vi "01 Dryer_Performance_SM.vi"() -> ()   [LabVIEW 2012]
uses:
  <vilib>/Platform/fileVersionInfo.llb/FileVersionInformation.ctl
  Equipment DPT.ctl
  WT500/Dryer PowerData.ctl
  Q Dryer Data.ctl
  DPT Global Type.ctl
  RMC Calc Inputs.ctl
  WT500/WT500 Sequences.ctl
  Chroma/Chroma Driver Select.ctl
  Dryer Wilt/Dryer Commands.ctl
  Nufi/Nufi Global_ReceivedDataCluster.vi
  Global Test Variables DPT.vi
  <vilib>/Analysis/baseanly.llb/Mean (DBL).vi
  <vilib>/Utility/file.llb/Write To Spreadsheet File (string).vi
  Drivers/Agilent 34970/Agilent 34970.lvlib
  <vilib>/Analysis/NI_AALBase.lvlib
panel:
  out "Low Power Switch":bool=TRUE
  out "Error Message 3":string
  out "Error Message 2":string
  in  "stop!":bool
  out "Tsamp(s)":dbl
  out "Temp OOR":bool
  in  "stop":bool
  in  "End Test Button":bool
  out "Data Filename":string
  in  "Tab Control":T1(tab)=enum."                           RMC  "
  in  "None":bool
  in  "All":bool
  out "Plot All":cluster{dbl[], dbl[]}[](graph)
  in  "Plot Legend":T2(array[cluster])
  out "2015?":bool
  out "Ave Gas Pressure":dbl format="%0.2f"
  out "Plot Power":cluster{dbl[], dbl[]}[](graph)
  out "PowerData":T3={"Current L1"=236.2, "Current L2"=17.749, "Power"=4192.0, "WattHours"=0.0}
  out "Power On":bool
  out "WH_0":dbl
  out "Wbouy":dbl
  out "Plot RMC":cluster{dbl[], dbl[]}[](graph)
  out "BDW - Bone Dry Wt(lbs)":dbl
  out "Empty Dryer Cold Weight":dbl
  out "Wet Clothing Weight":dbl
  out "Scale (LBS)":dbl
  out "RMC%":dbl=100.0
  out "Room Ambient F":dbl
  out "RDB F":dbl
  out "Cloth Weight(est.)":dbl
  out "Experimental Completion Time Estimate":dbl format="%<%H:%M:%S>t"
  out "Use Smoothing":bool=TRUE
  in  "Apply Load Offset":bool
  in  "Tab Control 2":enum32{"Debug Only", "Running"}(tab)
  in  "Debug Info":T4(tab)=enum."Settings"
  out "FileName DataLog":path caption="FileName"
  out "FileVersionInfo Out":T5
  out "Ver.":string="Development"
  out "Work File Directory":path=path "c:/Work"
  out "Number of TCs":i32
  in  "Close when complete":bool
  in  "DC Voltages Filename":path=path "c:/data/voltages.csv"
  out "Stream DC to File?":bool
  out "zip path":path
  out "Nufi Data File Path":path
  in  "Nufi?":bool=TRUE
  out "Filename Prefix String":string
  out "DOE Filename":path
  out "Error Log":errorcluster[](array[cluster])
  out "# elements in queue":i32
  out "Error Count":dbl
  out "error out":errorcluster
  out "Power Off Check":bool[](array[boolean])
  in  "Error Log 2":errorcluster[](array[cluster])
  out "Power Off Time(samples)":i32=15
  out "3011 resistor":dbl=267.4
  in  "UI Timer":i32=1000
  in  "DAQ Timer":i32=1000
  in  "Clear Graph":bool
  out "Use SL9200 Gas Readings?":bool
  in  "Simulate":bool
  in  "Supply Voltage:":string(combo)
  out "Equipment":T6
  out "Time Limit(s)":dbl=5400.0 format="%<%H:%M:%S>t"
  out "RMC Limit":dbl=2.0
  out "Enable Time Limit":bool
  out "Enable RMC Limit":bool
  in  "Weight Offset":dbl
  in  "MA Filter Size":i32=10
  in  "USB Weight?":bool=TRUE
  in  "Power On Threshold":dbl=50.0
  in  "Scale Temp Coeff":dbl
  out "Init Scale Temp":dbl=72.0
  out "3010 resistor":dbl=267.4
  out "Use Dry Gas Meter?":bool=TRUE
  out "Load Offset":dbl
  in  "Drum Volume":dbl=6.0
  out "Enable Stop On Power Off":bool=TRUE
  out "exe?":bool
  out "RMC Calc Inputs":T7
  out "Tend?":dbl format="%<%H:%M:%S>t"
  in  "W.Samps":i32=10
  out "1020 resistor":dbl=267.4
  in  "Auto Scale Reading":bool=TRUE
  out "Scale Com Port":refnum<visa-resource-name>="COM1"
  out "ITHX RH Sensor":bool
  out "Offset":dbl
  out "Init Offset Coeff":dbl
  in  "Power off Check RMC sec":dbl=7.0
  out "End4_Nufi":bool=TRUE
  out "Debug Mode":bool=TRUE
  out "Debug List Test States":string[](array[string])
  out "daq debug array":string[](array[string])
  out "UI States":string[](array[string])
  out "End1_Main":bool=TRUE
  out "Write to File":bool=TRUE
  out "Test Complete?":bool
  out "Loggin Data":bool
  out "End2_DAQ":bool=TRUE
  out "Eng3_Log":bool=TRUE
  out "BTUF3":string[][](array[string])
  out "Power On One Shot":bool
  out "Start Time (sec)":dbl format="%<%H:%M:%S>t"
  out "End Msg":string
  out "Final User Message":string="Premature Completion."
  out "cDAQ":bool=TRUE
  in  "cDAQ Setting":bool=TRUE
  out "End_End":bool=TRUE
  out "CDAQ Tasks":refnum<k21>[](array[refnum])
  out "[Temp (F), RH]":dbl[](array[numeric])
  out "Power Off One Shot":bool
  out "TC Chanel List":string
  out "DAQ Chanel List":string
  out "DAQ Label List":string[](array[string])
  out "Agilent Error Message":string
  out "DAQ Delay Time":i32
  in  "Get Data Interrupt":bool
  out "DAQ Data":dbl[](array[numeric])
  out "In Range?":bool[](array[boolean])
  in  "NPLC Value(6:1PLC)":T8(ring)=enum."1 PLC"
  in  "Channel Delay (sec)":dbl=0.01 format="%#_6e"
  in  "Channel Delay Auto (T:Enabled)":bool=TRUE
  in  "Autozero (0:ON)":enum16{"On", "Off", "Once"}(ring)
  in  "TC Check Enable (F:Disable)":bool=TRUE
  out "CDAQ Data Out":dbl[](array[numeric])
  out "Use Chroma":bool
  out "Globals for Dryer Performance Test":T9={"Test Setup"={"RH Resistor"=267.4, "Temp Cal"=72.0, "Temp Coeff"=-0.0234, "Power On Threshold"=50.0, "MA Filter Size"=60, "Weight Offset"=0.0, "Temp Resistor"=267.4, "Gas Enabled"=FALSE, "Gas P. Resistor"=250.0, "Scale Com"=1.0, "W. Samps"=5, "Temp4mA Val"=267.4, "Temp20mA Val"=267.4, "RH4mA Val"=0.0, "RH20mA Val"=100.0, "GPres4mA Val"=0.0, "Gpres20mA Val"=50.0, "Smoothing"=FALSE, "CDAQ"=FALSE, "34970"=FALSE, "34980"=FALSE, "RH-IP"="192.168.1.161", "RH-IP2"="192.168.1.161", "RH-IP3"="192.168.1.161", "CompVolume"=0.0, "T45_Coeff."=0.0}, "Agilent Setup"={"Scale Channel"="3009", "TC Channels"="1001:1040,2001:2040", "VDC Discrete Channels"="3001:3008", "RH Chan"="3010,3011", "Temp Chan"="3010,3011", "Tscale Channel"="", "RDB Channel"="1001", "Gas Temperature"="1019", "Gas Pressure"="1020", "Barometric Pressure"="1040", "Gas Feedback Chan"="3012"}, "Directories"={"Work File Directory"=path "c:/Work", "Save File Directory"=path "c:/Data", "Library Directory"=path "c:/Data", "Data Backup Directory"=path "c:/Data", "Data Backup Dir Fail"=path "c:/Data", "Lab Directory"=path "c:/Data"}, "Test Information"={"Model:"="DGnn", "Temperature:"="Mode: EHEAT", "Engineer:"="CraigT.", "Technician:"="RonR.", "Comments:"="R134A Charge Level: 50g", "Lab ID:"="DGnn", "TR Number:"="T000000", "Test Number:"="T000000", "Test Station:"="Unitialized", "Empty Dryer Cold Weight:"=0.0, "Serial Number:"="DGnn", "Build:"="DGnn", "Dryer Type"="RonR.", "Humidity"="70,50", "Test Title per TR:"="70,50"}, "cDAQ Array Locations"={"Scale Channel"="90", "TC Channels"="1-15, 65,66,67\n16-31, 68,69\n32-47, 70,71\n48-64, 72, 73", "VDC Discrete Channel"="1020,1040,3001:3008", "RH Chan"="91", "Temp Chan"="93", "Tscale Channel"="3", "RDB Channel"="1", "Gas Temperature"="0", "Gas Pressure"="89", "Barometric Pressure"="94", "Gas Feedback Chan"="92"}}
  out "Data":string[][](array[string])
  out "Power Label":string[](array[string])=["VL1", "VL2", "IL1", "IL2", "P", "WH", "Ipeak", "Phi(1,2)"]
  out "Q Element":T10
  in  "Start Test":bool
  out "Elapsed Time":dbl format="%<%H:%M:%S>t"
  out "Status Message":string
  # "Weight(Lbs)\nPower (Watts)\nCurrent (Amps)\nTemp(F)\nPressure (PSIA)\nRH (%)"
  # "(A)"
  # "(A)"
  # "(Watts)"
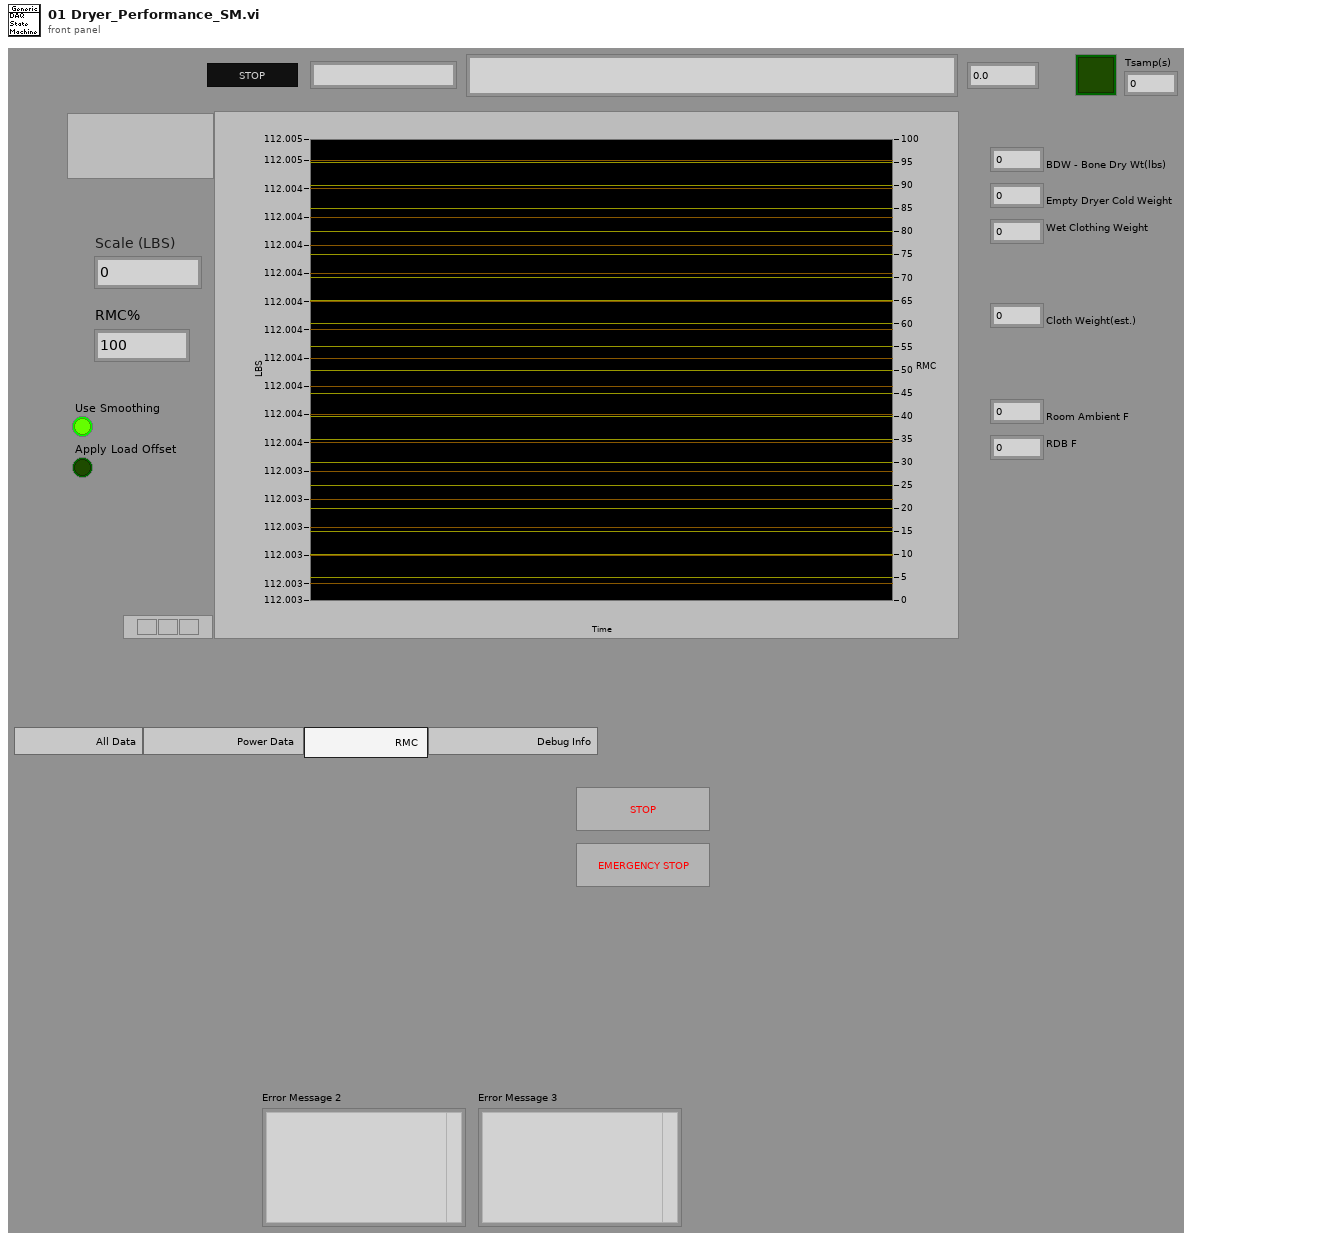
[diagram p1: front panel]
types:
  T1 = enum32{"                         All Data", "                            Power Data  ", "                           RMC  ", "                                  Debug Info"}
  T2 = cluster{"Title":string, "OnOff":bool, "Color Box":u32, "Value":dbl}[]
  T3 = typedef "Dryer PowerData.ctl" = cluster{"Current L1":dbl, "Current L2":dbl, "Power":dbl, "WattHours":dbl}
  T4 = enum32{"File Info", "Error Data", "Settings", "Test States", "Agilent Data", "Globals"}
  T5 = typedef "FileVersionInformation.ctl" = cluster{"FileVersion":string, "ProductName":string, "InternalName":string, "CompanyName":string, "LegalCopyright":string, "FileDescription":string}
  T6 = typedef "Equipment DPT.ctl" = cluster{"Com Agilent":refnum<visa-resource-name>, "Com Flow Computer":refnum<visa-resource-name>, "Com Power Meter":refnum<visa-resource-name>, "Com Power Supply":refnum<visa-resource-name>}
  T7 = typedef "RMC Calc Inputs.ctl" = cluster{"Measeured Weight":dbl, "BDW - Bone Dry Wt(lbs)":dbl, "Empty Dryer Cold Weight":dbl, "Measured IMC":dbl, "Tamb":dbl, "T-RDB":dbl, "Drum Volume":dbl, "Load Offset":dbl, "Temp Coeff":dbl, "Temp Cal":dbl, "Tscale":dbl}
  T8 = enum16{"0.02 PLC", "0.2 PLC", "1 PLC", "2 PLC", "10 PLC", "20 PLC", "100 PLC", "200 PLC"}
  T9 = typedef "DPT Global Type.ctl" = cluster{"Test Setup":cluster{"RH Resistor":dbl, "Temp Cal":dbl, "Temp Coeff":dbl, "Power On Threshold":dbl, "MA Filter Size":i32, "Weight Offset":dbl, "Temp Resistor":dbl, "Gas Enabled":bool, "Gas P. Resistor":dbl, "Scale Com":dbl, "W. Samps":i32, "Temp4mA Val":dbl, "Temp20mA Val":dbl, "RH4mA Val":dbl, "RH20mA Val":dbl, "GPres4mA Val":dbl, "Gpres20mA Val":dbl, "Smoothing":bool, "CDAQ":bool, "34970":bool, "34980":bool, "RH-IP":string, "RH-IP2":string, "RH-IP3":string, "CompVolume":dbl, "T45_Coeff.":dbl}, "Agilent Setup":cluster{"Scale Channel":string, "TC Channels":string, "VDC Discrete Channels":string, "RH Chan":string, "Temp Chan":string, "Tscale Channel":string, "RDB Channel":string, "Gas Temperature":string, "Gas Pressure":string, "Barometric Pressure":string, "Gas Feedback Chan":string}, "Directories":cluster{"Work File Directory":path, "Save File Directory":path, "Library Directory":path, "Data Backup Directory":path, "Data Backup Dir Fail":path, "Lab Directory":path}, "Test Information":cluster{"Model:":string, "Temperature:":string, "Engineer:":string, "Technician:":string, "Comments:":string, "Lab ID:":string, "TR Number:":string, "Test Number:":string, "Test Station:":string, "Empty Dryer Cold Weight:":dbl, "Serial Number:":string, "Build:":string, "Dryer Type":string, "Humidity":string, "Test Title per TR:":string}, "cDAQ Array Locations":cluster{"Scale Channel":string, "TC Channels":string, "VDC Discrete Channel":string, "RH Chan":string, "Temp Chan":string, "Tscale Channel":string, "RDB Channel":string, "Gas Temperature":string, "Gas Pressure":string, "Barometric Pressure":string, "Gas Feedback Chan":string}}
  T10 = typedef "Q Dryer Data.ctl" = cluster{"Data Array":dbl[], "Label Array":string[], "Date":string}
  T11 = enum32{"invalid app kind", "Development System", "Run Time System", "Student Edition", "Embedded LabVIEW", "Evaluation", "Custom"}
  T12 = typedef "WT500 Sequences.ctl" = enum16{"Initialize", "GetReadings", "GetErrors", "Close", "NoOp", "MiscCmd"}
  T13 = enum16{"DC Volts", "2-Wire Resistance", "4-Wire Resistance", "DC Current", "Temperature"}
  T14 = enum16{"B-Type", "E-Type", "J-Type", "K-Type", "N-Type", "R-Type", "S-Type", "T-Type"}
  T15 = enum16{"2252", "5000", "10000", "Default (Last)"}
  T16 = enum16{"100 mV", "1 V", "10 V", "100 V", "300 V", "Minimum", "Maximum"}
  T17 = cluster{"Thermocouple Type (Last)":enum16{"B", "E", "J", "K", "N", "R", "S", "T", "Default (Last)"}, "TC Rjunction (2:Int)":enum16{"Fixed", "External", "Internal"}, "Fixed Rjunction Temp (0:Manual)":enum16{"Manual", "Minimum", "Maximum"}, "TC Auto Check? (F:Don't Check)":bool, "Rjunct Temp Value (0)":dbl}
  T18 = enum16{"Exe", "Init CDAQ", "Gather DATA", "Close"}
  T19 = typedef "Chroma Driver Select.ctl" = enum16{"Initialize", "Output On 120", "Output On 240", "Output On 208", "Output Off", "Status", "Send Command", "Track Current"}
  T20 = enum16{"100 mV", "1 V", "10 V", "100 V", "300 V", "Auto", "Minimum", "Maximum", "Default"}
  T21 = enum32{"Invalid", "Standard", "Closed", "Hidden", "Minimized", "Maximized"}
  T22 = cluster{"Core":cluster{"Current VI Reference":refnum<vi>, "Close Panel on Exit?":bool}, "Error Log":errorcluster[], "FileName":path, "Config File Path":path, "Equipment":T6, "DAQ Chan List":string, "DAQ Label List":string[], "Supply Voltage:":string, "Empty Dryer Cold Weight":dbl, "Start Header Data":string[][], "Dryer Type":string, "Dryer Load Nominal Weight":string}
  T23 = typedef "DOE Audit Data.ctl" = cluster{"Technician":string, "Date":string, "Model":string, "Serial":string, "Total Dry Time(m)":dbl, "Bone Dry Wt":dbl, "Initial Wt":dbl, "Final Wt":dbl, "Initial Ret":dbl, "Final Ret":dbl, "Elect Energy Used":dbl, "Gas Meter Temp":dbl, "Gas Meter Pres":dbl, "Gas Volume":dbl, "Barometer Temp":dbl, "Barometer Pres":dbl, "Gas Corr Fact":dbl, "Cor Gas Vol":dbl, "Gas Heat Val":dbl, "Gas Energy BTU":dbl, "Gas Energy kwh 4%":dbl, "Elect Energy kwh 4%":dbl, "Total  Energy 4%":dbl, "Gas Vol Init":dbl, "Gas Vol Fin":dbl, "Start Time(s)":dbl, "End Time(s)":dbl, "Elect Energy Start":dbl, "Elect Energy End":dbl, "Per Cycle Efficency":dbl, "Annual Consumption":dbl, "Load Cycles":string, "Ambinet Temp":string, "Ambinet RH":string, "Per Cycle Off Mode/Standby Power":dbl, "Total Energy (Gas + Elect)":dbl, "Combined Energy Factor":dbl, "Off Mode Power":dbl, "Exhaust":string, "Washer Water Temperature ( 60 ± 5°F )":string, "Supply Voltage":string, "Reference Temperature (F)":string, "Reference Pressure (psi)":string, "Standby Power":dbl}
  T24 = enum16{"100 mV", "1 V", "10 V", "100 V", "300 V", "Auto", "Minimum", "Maximum"}
  T25 = typedef "Dryer Commands.ctl" = u8
  T26 = cluster{"[Temp (F), RH][0]":dbl, "[Temp (F), RH][1]":dbl}
  T27 = cluster{"Measured IMC":dbl, "Actual RMC":dbl, "RMC (Desired)":dbl, "Bone Dry Wt(lbs)":dbl, "Tolerance(%)":dbl}
  T28 = cluster{"Current VI Reference":refnum<vi>, "Close Panel on Exit?":bool}
  T29 = cluster{"queue out":refnum<queue>, "Q Element":T10, "Graph Reset":bool, "Init Save File":bool, "Time Array":dbl[], "Data Array":dbl[][], "Enable RMC":bool, "Power Previous":bool}
  T30 = cluster{"Title":string, "OnOff":bool, "Color Box":u32, "Value":dbl}
  T31 = cluster{"[0]":dbl, "[1]":dbl, "[2]":dbl, "[3]":dbl, "[4]":dbl, "[5]":dbl}
  T32 = cluster{"[0]":dbl, "[1]":dbl, "[2]":dbl, "[3]":dbl}
  T33 = enum16{"Left Button", "Center Button", "Right Button", "Window Close"}
  T34 = cluster{"queue out":refnum<queue>, "Q Element":T10, "Equipment":T6, "DAQ Chanel List":string, "Error Log 2":errorcluster[]}
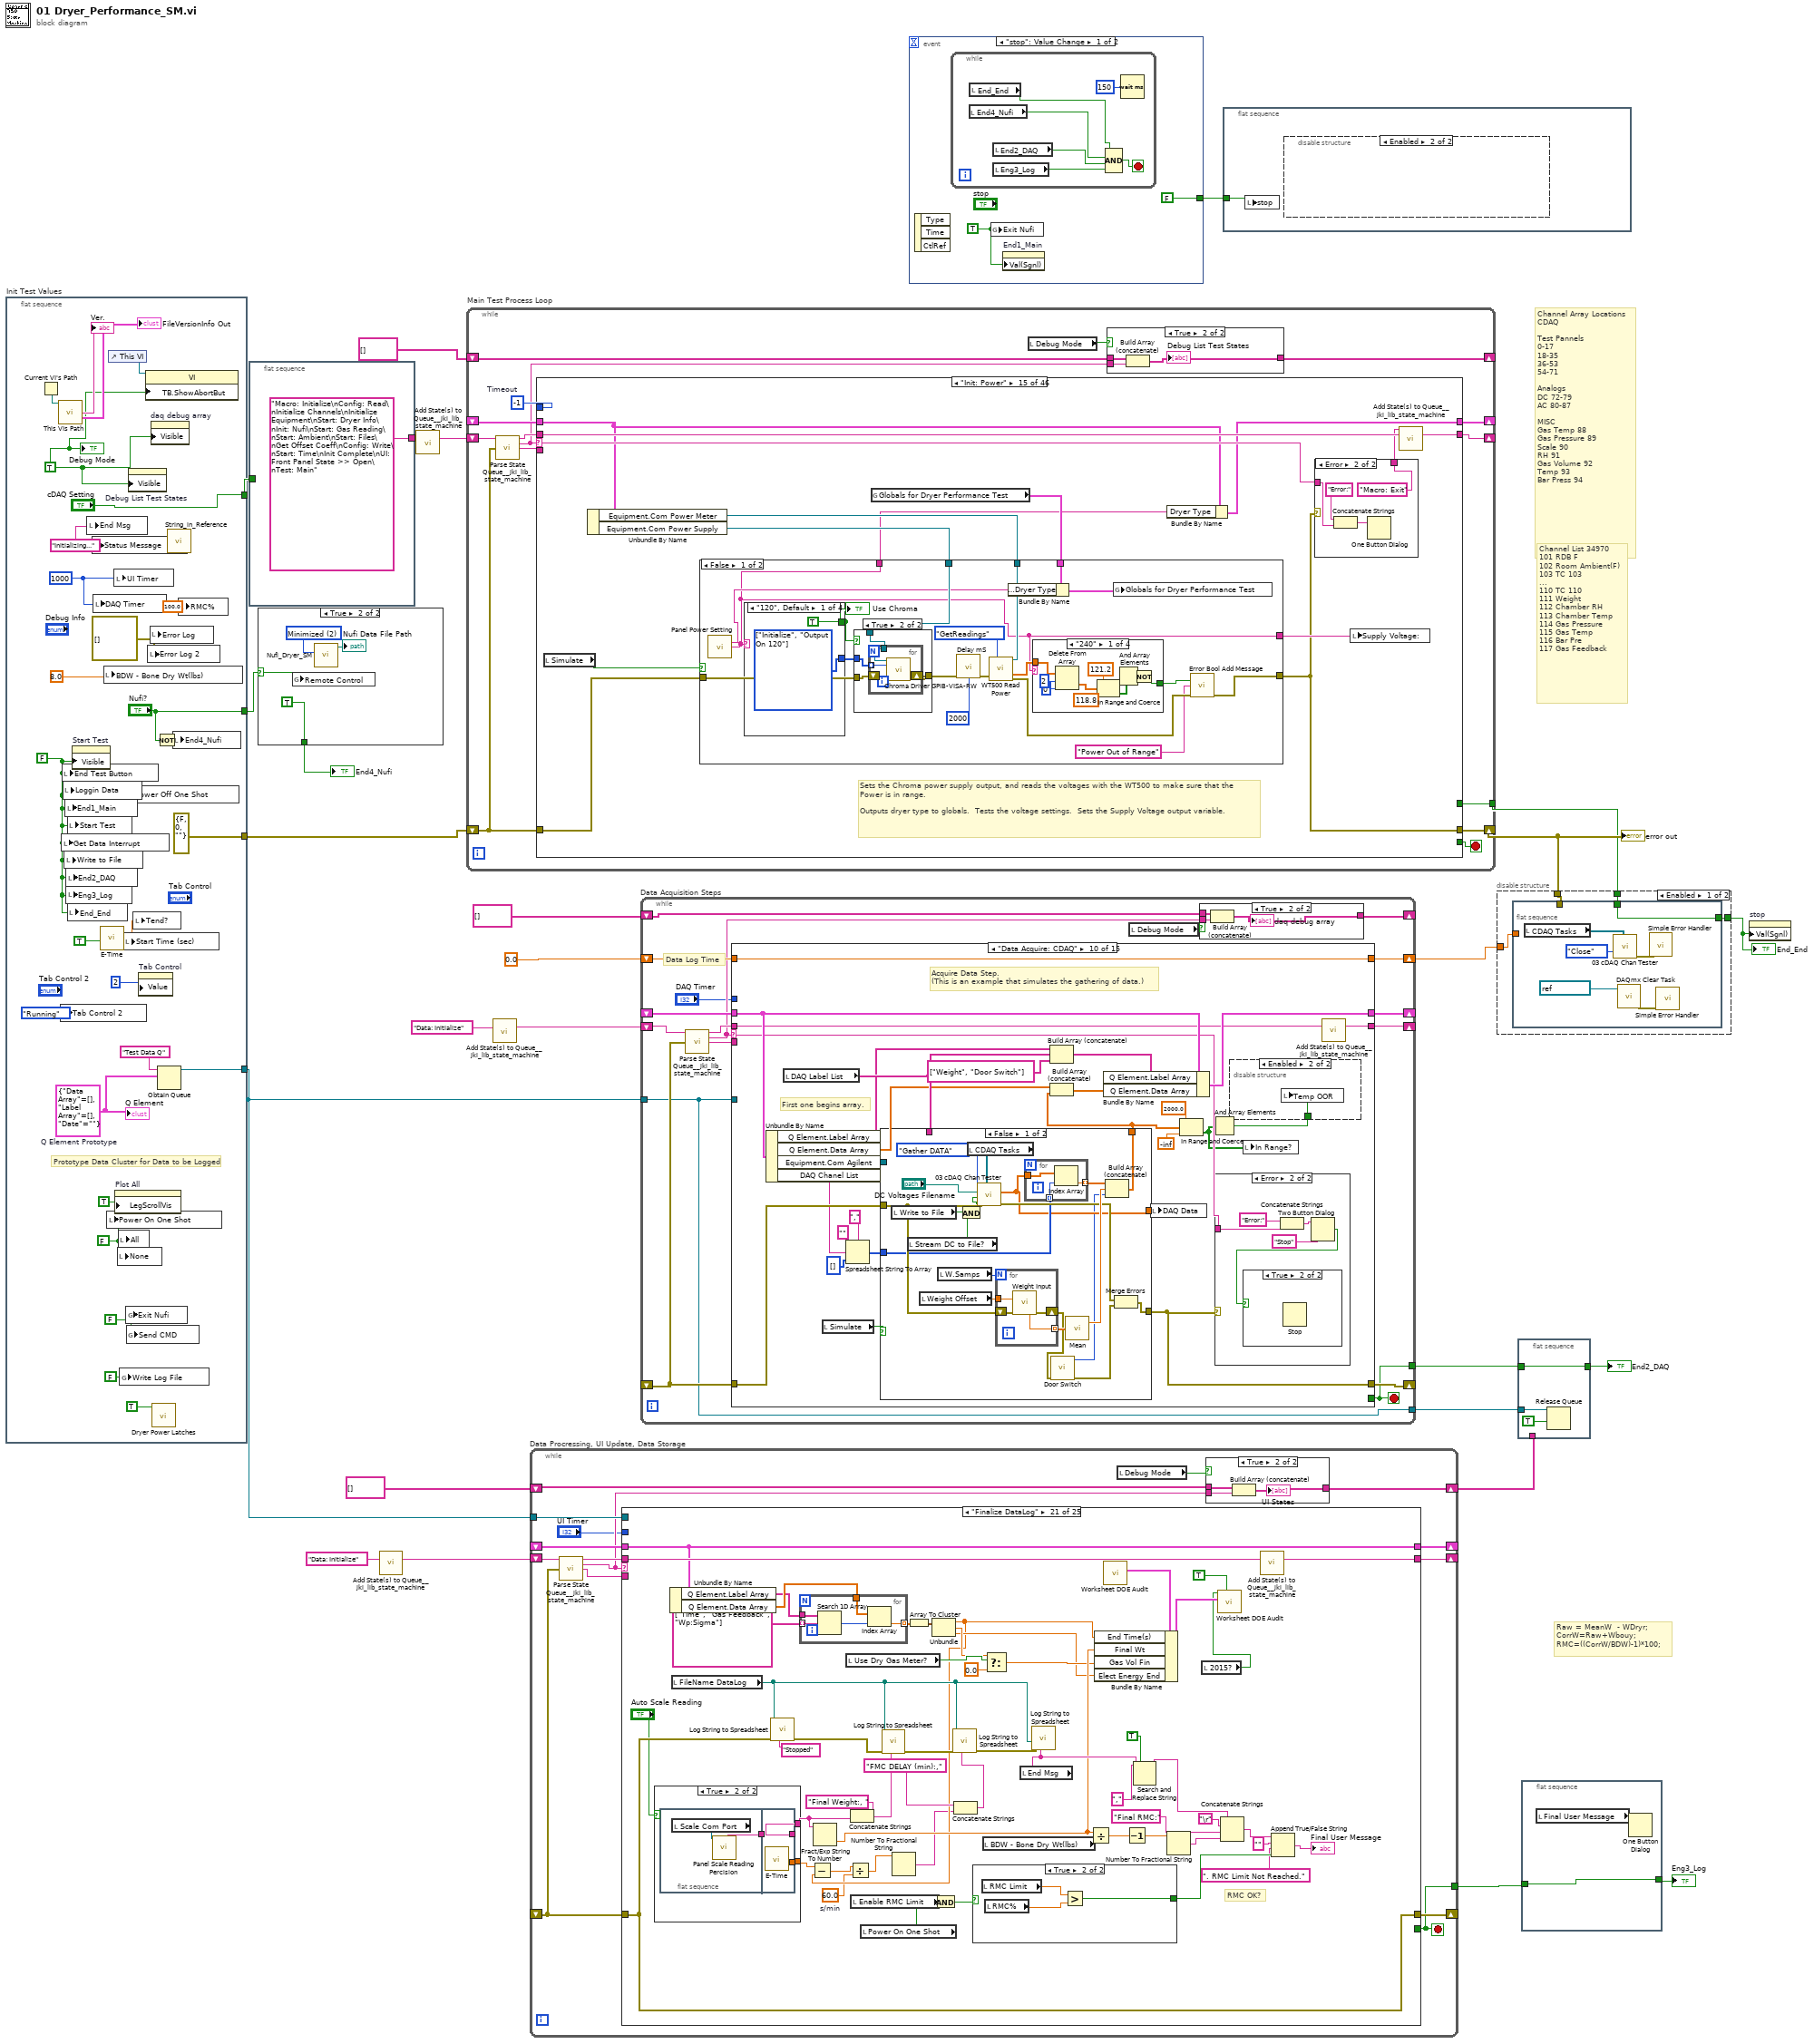
[diagram p0: block diagram]
diagram:
  # "Channel List 34970\n101 RDB F\n102 Room Ambient(F)\n103 TC 103\n...\n110 TC 110\n111 Weight\n112 Chamber RH\n113 Chamber Temp\n114 Gas Pressure\n115 Gas Temp\n116 Bar Pre\n117 Gas Feedback"
  # "Channel Array Locations\nCDAQ\n\nTest Pannels\n0-17\n18-35\n36-53\n54-71\n\nAnalogs\nDC 72-79\nAC 80-87\n\nMISC\nGas Temp 88\nGas Pressure 89\nScale 90\nRH 91\nGas Volume 92\nTemp 93\nBar Press 94"
  # "Raw = MeanW  - WDryr;\nCorrW=Raw+Wbouy;\nRMC=((CorrW/BDW)-1)*100;"
  n1 = flat-sequence "Init Test Values" {
    tunnel: [errorcluster {"status"=FALSE, "code"=0, "source"=""} ("Error Out")] -> w15
    tunnel: [w51] -> w23
    tunnel: ["cDAQ Setting"] -> w2
    tunnel: ["Nufi?"] -> w6
    frame #0 {
      w33 = FALSE ("Nufi Exit")
      w43 = FALSE ("Reset RMC")
      w34 = TRUE
      w49 = T10 {"Data Array"=[], "Label Array"=[], "Date"=""}  # Q Element Prototype
      w29 = errorcluster[] [] ("Error Log")
      w41 = "Initializing..." ("String")
      w48 = 1000 ("T1 ComTimer")
      w27 = FALSE ("Init Complete")
      # "Prototype Data Cluster for Data to be Logged"
      n2 = Current VI's Path() -> (path=w36:path)
      n3 = call "This VIs Path.vi"("path"=w36) -> ("File Version Info"=→"Ver.":string, "FileVersionInfo Out"=→"FileVersionInfo Out":T5)  [unwired: 10 in, 3 out]
      n4 = local write "Tab Control 2"(enum32{"Debug Only", "Running"}."Running" ("Tab Control 2")) -> ()
      n5 = local write "Get Data Interrupt"(w27) -> ()
      n6 = local write "End Test Button"(w27) -> ()
      n7 = local write "Loggin Data"(w27) -> ()
      n8 = local write "Write to File"(w27) -> ()
      n9 = local write "End1_Main"(w27) -> ()
      n10 = local write "End2_DAQ"(w27) -> ()
      n11 = local write "Eng3_Log"(w27) -> ()
      n12 = local write "Start Test"(w27) -> ()
      n13 = local write "End_End"(w27) -> ()
      n14 = property on="Start Test" class="Bool (strict)"("Visible"=w27) -> ()  [unwired: 2 in, 2 out]
      n15 = local write "End Msg"(w41) -> ()
      n16 = local write "Status Message"(w41) -> ()
      n17 = local write "DAQ Timer"(w48) -> ()
      n18 = call "E-Time.vi"("Reset"=TRUE) -> ("Elapsed Time (sec)"=w42:dbl)  [unwired: 8 in, 2 out]
      n19 = local write "BDW - Bone Dry Wt(lbs)"(8.0 ("BDW - Bone Dry Wt(lbs)")) -> ()
      n20 = local write "Power On One Shot"(w43) -> ()
      n21 = control-ref of="This VI"() -> (w44:refnum<vi>)
      n22 = local write "UI Timer"(w48) -> ()
      n23 = property on="Plot All" class="XYGraph (strict)"("LegScrollVis"=TRUE ("Legend:Scrollbar Visible")) -> ()  [unwired: 2 in, 2 out]
      n24 = local write "None"(w43) -> ()
      n25 = local write "All"(w43) -> ()
      n26 = global write "Nufi Global_ReceivedDataCluster.vi" "Write Log File"(FALSE ("Write Log File")) -> ()
      n27 = local write "Power Off One Shot"(w27) -> ()
      n28 = local write "Start Time (sec)"(w42) -> ()
      n29 = global write "Nufi Global_ReceivedDataCluster.vi" "Exit Nufi"(w33) -> ()
      n30 = global write "Nufi Global_ReceivedDataCluster.vi" "Send CMD"(w33) -> ()
      n31 = property on="Debug List Test States" class="Arr (strict)"("Visible"=w34) -> ()  [unwired: 2 in, 2 out]
      n32 = local write "Tend?"(w42) -> ()
      n33 = property on="Tab Control" class="TabCtl (strict)"("Value"=2) -> ()  [unwired: 2 in, 2 out]
      n34 = property class="VI"(reference=w44, "TB.ShowAbortBut"=w34) -> ()  [unwired: 1 in, 2 out]
      n35 = local write "Error Log 2"(w29) -> ()
      n36 = local write "Error Log"(w29) -> ()
      n37 = property on="daq debug array" class="Arr (strict)"("Visible"=w34) -> ()  [unwired: 2 in, 2 out]
      n38 = call "Dryer Power Latches.vi"("Init?"=TRUE) -> ()  [unwired: 8 in, 3 out]
      n39 = Not(x="Nufi?") -> (.not. x?=w30:bool)
      n40 = Obtain Queue(name (unnamed)="Test Data Q", element data type=w49) -> (queue out=w51:refnum<queue>)  [unwired: 3 in, 2 out]
      n41 = call "String_in_Reference.vi"("String"=w41) -> ()  [unwired: 18 in, 1 out]
      n42 = local write "End4_Nufi"(w30) -> ()
      n43 = local write "RMC%"(100.0 ("RMC")) -> ()
      "Q Element" <- w49
      "Debug Mode" <- w34
    }
  }
  n44 = flat-sequence {
    tunnel: ["Macro: Initialize\nConfig: Read\nInitialize Channels\nInitialize Equipment\nStart: Dryer Info\nInit: Nufi\nStart: Gas Reading\nStart: Ambient\nStart: Files\nGet Offset Coeff\nConfig: Write\nStart: Time\nInit Complete\nUI: Front Panel State >> Open\nTest: Main"] -> w13
    tunnel: w2 -> [_]
    frame #0 {
    }
  }
  n45 = case shown="True" w6 {
    selector: w6 -> [_ w56]
    tunnel: [TRUE ("Finish") TRUE ("Finish")] -> w1
    frame False {
    }
    frame True {
      w58 = u16 2 items=["Open", "Closed", "Minimized"] ("Front Panel")
      n46 = global write "Nufi Global_ReceivedDataCluster.vi" "Remote Control"(w56) -> ()
      n47 = call "Nufi_Dryer_SM.vi"("Front Panel"=w58) -> ("Saved Filename Out"=→"Nufi Data File Path":path)  [unwired: 10 in]
    }
  }
  "End4_Nufi" <- w1
  n48 = call <vilib>:"Add State(s) to Queue__jki_lib_state_machine.vi"("State(s) in (\"\")"="Data: Initialize") -> ("States Out"=w4:string)  [unwired: 14 in]
  n49 = call <vilib>:"Add State(s) to Queue__jki_lib_state_machine.vi"("State(s) in (\"\")"=w13) -> ("States Out"=w19:string)  [unwired: 14 in]
  n50 = while "Main Test Process Loop" {
    shift-right: [w70] -> _
    shift-left: _ -> [w69]
    shift-right: [w72] -> w10
    shift-left: w15 -> [w67]
    shift-right: [w71] -> _
    shift-left: w19 -> [w73]
    shift-right: [w65] -> _
    shift-left: string[] [] -> [w64]
    tunnel: [w60] -> w7
    stop <- w66 stop-if-true
    w68 = -1  # Timeout
    n51 = call <vilib>:"Parse State Queue__jki_lib_state_machine.vi"("State Queue"=w73, "Error In (no error)"=w67) -> ("Remaining States"=w74:string, "Current State"=w62:string, "Arguments"=w63:string)  [unwired: 11 in]
    n52 = case shown="\"Init: Power\"" w62 {
      selector: w62 -> [_ _ _ w113 _ _ _ _ _ _ _ _ _ _ w464 w555 w581 w619 w730 _ _ _ _ w850 w912 w977 w1090 _ _ _ _ _ _ _ _ _ _ _ _ _ _ _ _ _ _ w1396]
      tunnel: w74 -> [w80 w88 w112 w117 w133 w155 w159 w171 w182 w229 w286 w370 w400 w432 w472 w560 w589 w626 w737 w813 w818 w831 w837 w853 w915 w980 w1097 w1136 w1159 w1167 w1183 w1193 w1218 w1226 w1255 w1269 w1277 w1281 w1286 w1303 w1307 w1328 w1386 w1391 w1395 w1404]
      tunnel: w63 -> [_ _ _ _ _ _ _ _ _ _ _ _ _ _ _ _ _ _ _ _ _ _ _ _ _ _ _ _ _ _ _ _ _ w1220 _ _ _ _ _ _ _ _ _ _ _ _]
      tunnel: w69 -> [w81 w86 w109 w115 w129 w153 w156 w162 w179 w226 w283 w367 w397 w428 w461 w554 w587 w620 w731 w811 w816 w828 w834 w846 w909 w974 w1088 w1133 w1156 w1164 _ w1191 w1215 w1222 w1252 w1267 w1275 w1278 w1283 w1300 w1304 w1324 w1384 w1389 w1392 w1402]
      tunnel: [w79 w85 w110 w119 errorcluster {"status"=FALSE, "code"=0, "source"=""} ("error out") w151 w157 w168 w180 w227 w284 w368 w398 w422 w466 w557 w583 w621 w732 w806 w815 w829 w835 w847 w907 w972 w1072 w1132 w1157 w1165 w1178 w1188 w1216 w1223 w1253 w1265 w1272 w1279 w1284 w1301 w1305 w1326 w1383 w1388 w1393 w1398] -> w72
      tunnel: w67 -> [w79 w84 w110 w118 w126 w151 w157 w168 w180 w227 w284 w368 w398 w423 w467 w558 w584 w622 w733 w809 w815 w829 w835 w849 w911 w976 w1081 w1132 w1157 w1165 w1178 w1189 w1216 w1224 w1253 w1266 w1273 w1279 w1284 w1301 w1305 w1326 w1383 w1388 w1393 w1399]
      tunnel: [w80 w87 w111 w116 w132 w154 w158 w170 w181 w228 w285 w369 w399 w431 w471 w559 w588 w625 w736 w812 w817 w830 w836 w852 w914 w979 w1096 w1135 w1158 w1166 w1182 w1192 w1217 w1225 w1254 w1268 w1276 w1280 w1285 w1302 w1306 w1327 w1385 w1390 w1394 w1403] -> w71
      tunnel: [_ _ _ _ _ w150 _ _ _ _ _ _ _ _ _ _ _ _ _ _ _ _ _ _ _ _ _ _ _ _ _ _ _ _ _ _ _ _ _ _ _ _ _ _ _ _] -> w66
      tunnel: [w81 w83 w109 w115 w128 w153 w156 w169 w179 w225 w282 w366 w397 w427 w460 w553 w587 w620 w731 w811 w816 w828 w834 w845 w908 w973 w1064 w1133 w1156 w1164 w1181 w1191 w1215 w1222 w1252 w1267 w1275 w1278 w1283 w1300 w1304 w1324 w1384 w1389 w1392 w1402] -> w70
      tunnel: w68 -> [_ w82 _ _ _ _ _ _ _ _ _ _ _ _ _ _ _ _ _ _ _ _ _ _ _ _ _ _ _ _ _ _ _ _ _ _ _ _ _ _ _ _ _ _ _ _]
      tunnel: [_ _ _ _ _ w150 _ _ _ _ _ _ _ _ _ _ _ _ _ _ _ _ _ _ _ _ _ _ _ _ _ _ _ _ _ _ _ _ _ _ _ _ _ _ _ _] -> w60
      frame "ABOUT" {
        (unwired) "This Program has 3 state machines.  The top is the main test loop, where the test sequence is executed. The Second is the Data Acquisition state machine.  It puts the data into a Q that has the datat titles, and raw data in it.  The third \nState Machine deques the Q, saving, processing and displaying the Data.\n\nLegacy code for Agilent still remains.  CDAQ is the main daq."
      }
      frame "", "Idle" {
        # "executes when the state queue is empty"
        n53 = event shown="[1] \"End Test Button\": Value Change" {
          selector: _ -> [_ _ _ _]
          dyn-events: _ -> [_ _ _ _]
          timeout: w82 -> [_ _ _ _]
          tunnel: w88 -> [w92 w97 w102 w108]
          tunnel: [w91 w96 w101 w107] -> w87
          tunnel: w86 -> [w89 w94 w99 w105]
          tunnel: [w90 w95 w100 w106] -> w85
          tunnel: w84 -> [w90 w95 w100 w106]
          tunnel: [w89 w94 w99 w105] -> w83
          event Timeout {
            n54 = event-data() -> ()  [unwired: 1 in, 1 out]
            n55 = call <vilib>:"Add State(s) to Queue__jki_lib_state_machine.vi"("State(s) in (\"\")"=w92) -> ("States Out"=w91:string)  [unwired: 14 in]
          }
          event "End Test Button": Value Change {
            # "Exit Button Value Change (pressed) Event\n(this executes Macro: Exit to terminate the VI)"
            n56 = event-data() -> ()  [unwired: 1 in, 1 out]
            n57 = call <vilib>:"Add State(s) to Queue__jki_lib_state_machine.vi"("State(s) in Front (\"\")"="Power Off\nMacro: Exit", "State(s) in (\"\")"=w97) -> ("States Out"=w96:string)  [unwired: 13 in]
          }
          event "Start Test": Value Change {
            # "This will stop logging until the test is running."
            n58 = event-data() -> ()  [unwired: 1 in, 6 out]
            n59 = call <vilib>:"Add State(s) to Queue__jki_lib_state_machine.vi"("State(s) in Front (\"\")"="Start: Dryer Info\nStart: Gas Reading\nStart: Files\nConfig: Write\nStart: Time\nTest: Main", "State(s) in (\"\")"=w102) -> ("States Out"=w101:string)  [unwired: 13 in]
          }
          event Panel Close? {
            # "Discard the event because we'll close the front panel ourselves in Macro: Exit"
            # "Close Panel button (pressed) Event\n(this executes Macro: Exit to terminate the VI)"
            n60 = event-data() -> ()  [unwired: 1 in, 1 out]
            n61 = call <vilib>:"Add State(s) to Queue__jki_lib_state_machine.vi"("State(s) in Front (\"\")"="Macro: Exit", "State(s) in (\"\")"=w108) -> ("States Out"=w107:string)  [unwired: 13 in]
            n62 = event-data("Discard?"=TRUE) -> ()  [unwired: 1 in, 1 out]
          }
        }
      }
      frame "---------- Core ----------" {
        # "Do not put any code in this frame.\n(it is a separator no-op)"
        n63 = call <vilib>:"Add State(s) to Queue__jki_lib_state_machine.vi"("State(s) in (\"\")"=w112) -> ("States Out"=w111:string)  [unwired: 14 in]
      }
      frame Default {
        w122 = 42 items=["No error", "Argument error", "Memory is full", "Out of zone", "End of file", "File already open", "Generic file I/O error", "File not found", "File permission error", "Disk is full", "Duplicate path", "Too many files open", "System feature not enabled", "Resource file not found", "Cannot add resource", "Resource not found", "Image not found", "Image memory error", "Pen does not exist", "Config type invalid", "Config token not found", "Config parse error", "Config memory error", "Bad external code format", "Bad external code offset", "External code not present", "Null window", "Destroy window error", "Null menu", "Print aborted", "Bad print record", "Print driver error", "Windows error during printing", "Memory error during printing", "Print dialog error", "Generic print error", "Invalid device refnum", "Device not found", "Device parameter error", "Device unit error", "Cannot open device", "Device call aborted", "Generic error", "Cancelled by user", "Object ID too low", "Object ID too high", "Object not in heap", "Unknown heap", "Unknown object (invalid DefProc)", "Unknown object (DefProc not in table)", "Message out of range", "Invalid (null) method", "Unknown message", "Manager call not supported", "Bad address", "Network operation in progress", "Network operation timed out", "Connection is busy", "Network attribute not supported", "Network error", "Address in use", "System out of memory", "Connection aborted", "Connection refused", "Not connected", "Already connected", "Connection closed", "Initialization error (interapplication manager)", "Bad occurrence", "Wait on unbound occurrence handler", "Occurrence queue overflow", "Datalog type conflict", "Unused", "Unrecognized type (interapplication manager)", "Memory corrupt", "Failed to make temporary DLL", "Old CIN version", "Drag socket not found", "Failed to load drop-object", "Failed to register OLE object", "Failed to release OLE object", "Format specifier type mismatch", "Unknown format specifier", "Too few format specifiers", "Too many format specifiers", "Scan failed", "Newer CIN version", "Error converting to variant", "Runtime menu error", "Password tampered", "Variant attribute not found", "Incompatible variant data type", "Event data is not available", "Event Store is not present", "Occurrence is not found", "Event Queue is not created", "Event info is not available", "Refnum passed is NULL", "Error retrieving Class GUID", "Error retrieving CoClass GUID", "Error retrieving TypeLib GUID.", "Bad built application magic bytes.", "Specific driver is different from the specific driver associated with the Logical Name.", "There is no session opened to the class driver.", "Max Error", "MAX - Error with config objects", "MAX - Error loading configuration", "MAX - Group not supported"]
        # "Current State"
        # "Do not delete, rename, or modify this frame.\n(this is used to capture unhandled states and typos)"
        # "Handle mistyped state name (developer tool)"
        n64 = Format Into String(format string="Software Exception: Unhandled State \"%s\"." ("message"), error in=w118, w113) -> (resulting string=w121:string, error out=w120:errorcluster)  [unwired: 1 in]
        n65 = call <vilib>:"Error Cluster From Error Code.vi"("show call chain? (False)"=TRUE, "error in (no error)"=w120, "error message (\"\")"=w121, "error code (0)"=w122) -> ("error out"=w119:errorcluster)  [unwired: 5 in]
        n66 = call <vilib>:"Add State(s) to Queue__jki_lib_state_machine.vi"("State(s) in (\"\")"=w117) -> ("States Out"=w116:string)  [unwired: 14 in]
      }
      frame "Error Handler" {
        # "Unhandled Error -- Display it"
        # "Handle any errors here.\nYou can also output any states to clean-up after errors occur"
        # "Clear error"
        n67 = Unbundle By Name(w129) -> ("Error Log"=w130:errorcluster[])
        n68 = local read "Loggin Data"() -> (w125:bool)
        n69 = Build Array (concatenate)(w130, w126) -> (w127:errorcluster[])
        n70 = case shown="False" w125 {
          tunnel: w127 -> [w134 w147]
          tunnel: w126 -> [_ w146]
          tunnel: ["Macro: Exit" "Macro: Exit"] -> w124
          frame False {
            n71 = local write "Error Log"(w134) -> ()
          }
          frame True {
            n72 = call "Counter.vi"() -> ("Count"=w144:dbl)  [unwired: 11 in]
            "Error Count" <- w144
            n73 = Unbundle By Name(w146) -> ("code"=w139:i32, "source"=w140:string)  [unwired: 1 out]
            n74 = local read "Write to File"() -> (w136:bool)
            n75 = Format Into String(format string="%s %d %s %d %s %s", "Error Count: " ("input 1"), w144, " Code: " ("input 1"), w139, " Source: " ("input 1"), w140) -> (resulting string=w138:string)  [unwired: 2 in, 1 out]
            n76 = case shown="True" w136 {
              tunnel: w138 -> [_ w149]
              frame False {
              }
              frame True {
                n77 = local read "FileName DataLog"() -> (w148:path)
                n78 = call "Log String to Spreadsheet.vi"("String"=w149, "FileName"=w148) -> ()  [unwired: 9 in, 1 out]
              }
            }
            "Error Log" <- w147
          }
        }
        n79 = Bundle By Name(cluster=w129, "Error Log"=w127) -> (w128:T22)
        n80 = call <vilib>:"Add State(s) to Queue__jki_lib_state_machine.vi"("State(s) in Front (\"\")"=w124, "State(s) in (\"\")"=w133) -> ("States Out"=w132:string)  [unwired: 13 in]
      }
      frame "Exit" {
        w150 = TRUE
        # "Do not put any code in this frame.\n(No errors that occur here will be handled.)"
        n81 = call "String_in_Reference.vi"("String"="Stopping Test..." ("string")) -> ()  [unwired: 18 in, 1 out]
        n82 = call <vilib>:"Add State(s) to Queue__jki_lib_state_machine.vi"("State(s) in (\"\")"=w155) -> ("States Out"=w154:string)  [unwired: 14 in]
      }
      frame "-------Initialize-------" {
        # "Do not put any code in this frame.\n(It is a separator no-op. You can make a copy of this frame to create a new Data frame)"
        n83 = call <vilib>:"Add State(s) to Queue__jki_lib_state_machine.vi"("State(s) in (\"\")"=w159) -> ("States Out"=w158:string)  [unwired: 14 in]
      }
      frame "Initialize Core Data" {
        # "Do not delete, rename, or modify this frame.\n(this is used to determine panel behavior on exit)"
        # "originally closed?"
        # "exe?"
        # "If panel starts closed or is an EXE, then close it when we exit"
        n84 = property class="VI"() -> ("Front Panel.Open"=w167:bool)  [unwired: 2 in, 2 out]
        n85 = control-ref of="Current VI Reference"() -> (w160:refnum<vi>)
        n86 = property class="App"() -> ("App.Kind"=w166:T11)  [unwired: 2 in, 2 out]
        n87 = Not(x=w167) -> (.not. x?=w164:bool)
        n88 = Equal?(x=w166, y=T11."Run Time System" ("Application:Kind")) -> (x = y?=w163:bool)
        "exe?" <- w163
        n89 = Or(x=w164, y=w163) -> (x .or. y?=w161:bool)
        n90 = Bundle By Name(cluster=w162, "Core.Current VI Reference"=w160, "Core.Close Panel on Exit?"=w161) -> (w169:T22)
        n91 = call <vilib>:"Add State(s) to Queue__jki_lib_state_machine.vi"("State(s) in (\"\")"=w171) -> ("States Out"=w170:string)  [unwired: 14 in]
      }
      frame "Initialize Channels" {
        # "4"
        n92 = global read "Global Test Variables DPT.vi" "Globals for Dryer Performance Test"() -> (w177:T9)
        n93 = Unbundle By Name(w177) -> ("Test Setup.CDAQ"=w176:bool, "Test Setup.34970"=w175:bool, "Test Setup.34980"=w174:bool)
        n94 = Build Array(w176, w175, w174) -> (w173:bool[])
        n95 = Boolean Array To Number(Boolean array=w173) -> (number=w172:u32)
        n96 = case shown="4" w172 {
          tunnel: ["Initialize CDAQ Channels" ("State(s) in Front (\"\")") "Initialize 34970 Channels" ("State(s) in Front (\"\")") "Initialize Agilent Channels" ("State(s) in Front (\"\")")] -> w178
          frame 1, Default {
          }
          frame 2 {
          }
          frame 4 {
          }
        }
        n97 = call <vilib>:"Add State(s) to Queue__jki_lib_state_machine.vi"("State(s) in Front (\"\")"=w178, "State(s) in (\"\")"=w182) -> ("States Out"=w181:string)  [unwired: 13 in]
      }
      frame "Initialize Agilent Channels" {
        # "if ends in , remove it"
        n98 = global read "Global Test Variables DPT.vi" "Globals for Dryer Performance Test"() -> (w201:T9)
        n99 = local read "cDAQ"() -> (w186:bool)
        n100 = Unbundle By Name(w201) -> ("Agilent Setup.Scale Channel"=w200:string, "Agilent Setup.RH Chan"=w199:string, "Agilent Setup.Temp Chan"=w198:string, "Agilent Setup.Gas Feedback Chan"=w187:string, "Test Setup.Gas Enabled"=w197:bool, "Agilent Setup.Gas Pressure"=w196:string, "Agilent Setup.Gas Temperature"=w195:string, "Agilent Setup.Barometric Pressure"=w194:string)
        n101 = call "Panel DPT Channel Test Labels.vi"("CDAQ?"=w186) -> ("Chanel List"=w208:string, "Label Array"=w217:string[])  [unwired: 12 in, 1 out]
        "TC Chanel List" <- w208
        n102 = local read "USB Weight?"() -> (w202:bool)
        n103 = Search and Replace String(replace all?=TRUE ("replace all? (F)"), input string=w208, search string=",") -> (number of replacements=w205:i32)  [unwired: 5 in, 3 out]
        n104 = Increment(x=w205) -> (x+1=→"Number of TCs":i32)
        n105 = call "Panel DPT Voltage Labels.vi"("Chanel List In"=w208, "CDAQ?"=w186, "Label List In"=w217) -> ("Chanel List Out"=w218:string, "Label List Out"=w216:string[])  [unwired: 10 in, 1 out]
        n106 = case shown="True" w202 {
          tunnel: [string[] ["Weight", "Chamber RH", "Chamber Temp"] ("Label List 2") string[] ["Agilent Weight", "Chamber RH", "Chamber Temp"] ("Label List 2")] -> w224
          tunnel: [w243 w249] -> w203
          tunnel: w200 -> [w242 w248]
          tunnel: w199 -> [w241 w247]
          tunnel: w198 -> [w240 w246]
          frame False {
            w239 = "," ("string")
            n107 = Concatenate Strings(w242, w239, w241, w239, w240) -> (w243:string)
          }
          frame True {
            w245 = "," ("string")
            n108 = Concatenate Strings(w248, w245, w247, w245, w246) -> (w249:string)
          }
        }
        n109 = String Length(string=w218) -> (length=w223:i32)
        n110 = Greater Than 0?(x=w223) -> (x > 0?=w220:bool)
        n111 = Select(t=",", s=w220, f="") -> (s? t:f=w219:string)
        n112 = case shown="True" w197 {
          tunnel: w196 -> [_ w238]
          tunnel: w195 -> [_ w237]
          tunnel: w194 -> [_ w236]
          tunnel: ["" w235] -> w193
          tunnel: [string[] [] ("Label List 2") string[] ["Gas Pressure", "Gas Temperature", "Barometric Pressure", "Gas Feedback"] ("Label List 2")] -> w192
          tunnel: w187 -> [_ w232]
          frame False {
          }
          frame True {
            w233 = "," ("string")
            n113 = Concatenate Strings(w233, w238, w233, w237, w233, w236, w233, w232) -> (w235:string)
          }
        }
        n114 = Concatenate Strings(w218, w219, w203, w193) -> (w210:string)
        n115 = Build Array (concatenate)(w216, w224, w192) -> (w189:string[])
        n116 = String Length(string=w210) -> (length=w215:i32)
        n117 = Decrement(x=w215) -> (x-1=w209:i32)
        n118 = String Subset(string=w210, offset (0)=w209, length (rest)=1 ("length (rest)")) -> (substring=w213:string)
        n119 = Equal?(x=w213, y=",") -> (x = y?=w211:bool)
        n120 = case shown="True" w211 {
          tunnel: w210 -> [w251 w255]
          tunnel: w209 -> [_ w253]
          tunnel: [w251 w252] -> w191
          frame False {
          }
          frame True {
            n121 = String Subset(string=w255, offset (0)=0, length (rest)=w253) -> (substring=w252:string)
          }
        }
        n122 = call "Agilent Sort Channels.vi"("Agilent Chanel List"=w191, "Agilent Label List"=w189) -> ("Sorted Channels"=w190:string, "Sorted Labels Array"=w188:string[])  [unwired: 12 in]
        "DAQ Chanel List" <- w190
        "DAQ Label List" <- w188
        n123 = Bundle By Name(cluster=w226, "DAQ Chan List"=w190, "DAQ Label List"=w188) -> (w225:T22)
        n124 = call <vilib>:"Add State(s) to Queue__jki_lib_state_machine.vi"("State(s) in (\"\")"=w229) -> ("States Out"=w228:string)  [unwired: 14 in]
      }
      frame "Initialize 34970 Channels" {
        # "FIXME: ALL MAGIC NUM CONFIG"
        # "Assume no gas, since not set up for 34970"
        # "if ends in , remove it"
        n125 = global read "Global Test Variables DPT.vi" "Globals for Dryer Performance Test"() -> (w265:T9)
        n126 = disable-structure shown="Enabled" {
          disable-tunnel: [w292 ","] -> w280
          disable-tunnel: [w291 w298] -> w279
          disable-tunnel: [w289 w299] -> w278
          disable-tunnel: [w287 w298] -> w258
          frame Disabled {
            n127 = local read "cDAQ"() -> (w288:bool)
            n128 = call "Panel DPT Channel Test Labels.vi"("CDAQ?"=w288) -> ("Chanel List"=w287:string, "Label Array"=w290:string[])  [unwired: 12 in, 1 out]
            n129 = call "Panel DPT Voltage Labels.vi"("Chanel List In"=w287, "CDAQ?"=w288, "Label List In"=w290) -> ("Chanel List Out"=w291:string, "Label List Out"=w289:string[])  [unwired: 10 in, 1 out]
            n130 = String Length(string=w291) -> (length=w296:i32)
            n131 = Greater Than 0?(x=w296) -> (x > 0?=w293:bool)
            n132 = Select(t=",", s=w293, f="") -> (s? t:f=w292:string)
          }
          frame Enabled {
            n133 = global read "Global Test Variables DPT.vi" "34970 TC Chan List"() -> (w298:string)
            n134 = global read "Global Test Variables DPT.vi" "34970 Label List"() -> (w299:string[])
          }
        }
        n135 = Unbundle By Name(w265) -> ("Test Setup.Gas Enabled"=w264:bool)
        n136 = local write "TC Chanel List"(w258) -> ()
        n137 = local read "USB Weight?"() -> (w266:bool)
        n138 = Search and Replace String(replace all?=TRUE ("replace all? (F)"), input string=w258, search string=",") -> (number of replacements=w268:i32)  [unwired: 5 in, 3 out]
        n139 = Increment(x=w268) -> (x+1=w257:i32)
        n140 = local write "Number of TCs"(w257) -> ()
        n141 = case shown="False" w266 {
          tunnel: [string[] ["Weight", "Chamber RH", "Chamber Temp"] ("Label List 2") string[] ["Agilent Weight", "Chamber RH", "Chamber Temp"] ("Label List 2")] -> w281
          tunnel: [w313 w319] -> w267
          frame False {
            w312 = "," ("string")
            n142 = Concatenate Strings("111" ("string"), w312, "112" ("string"), w312, "113" ("string")) -> (w313:string)
          }
          frame True {
            w318 = "," ("string")
            n143 = Concatenate Strings("111" ("string"), w318, "112" ("string"), w318, "113" ("string")) -> (w319:string)
          }
        }
        n144 = case shown="True" w264 {
          tunnel: ["" w308] -> w263
          tunnel: [string[] [] ("Label List 2") string[] ["Gas Pressure", "Gas Temperature", "Barometric Pressure", "Gas Feedback"] ("Label List 2")] -> w262
          frame False {
          }
          frame True {
            w306 = "," ("string")
            n145 = Concatenate Strings(w306, "114" ("string"), w306, "115" ("string"), w306, "116" ("string"), w306, "117" ("string")) -> (w308:string)
          }
        }